vi "UHR-Fleezers Control (host) - 12.6.1.vi"() -> ()   [LabVIEW 2012] (continued)
  T22 = cluster{"New Image":T2, "New Image":T2, "New Image":T2, "New Image":T2, "New Image":T2}
  T23 = typedef "XDNodeRunTimeDep.lvlib/timing_clust.ctl" = cluster{"Expected End [f-1]":u64, "Actual End [f-1]":u64, "Finished Late? [f-1]":bool, "Expected End [i-1]":u64, "Actual End [i-1]":u64, "Finished Late? [i-1]":bool, "Expected Start [i]":u64, "Actual Start [i]":u64, "Expected Start [f]":u64, "Actual Start [f]":u64, "Source Name":string, "Structure Name":string, "Period":i64, "Deadline":i64, "Offset":i64, "Start":i64, "Priority":i32, "Timeout":i32, "Mode":T24, "Wakeup Reason":T25, "Error":errorcluster, "Source Type":string, "Secondary Source Type":string, "Global End Time":u64, "Global Start Time":u64, "Frame Duration":u64, "Iteration Duration":u64, "Assigned CPU":i32, "I/O Scan Engine Mode":u32}
  T24 = typedef "XDNodeRunTimeDep.lvlib/nitl_modes.ctl" = enum32{"No Change", "Process missed periods, maintain original phase", "Discard missed periods, maintain original phase", "Process missed periods, ignore original phase", "Discard missed periods, ignore original phase"}
  T25 = typedef "XDNodeRunTimeDep.lvlib/wakeup.ctl" = enum32{"Normal", "Aborted", "Asynchronous wakeup", "Timing source error", "Timed loop error", "Timeout"}
  T26 = enum32{"Status", "Sample Stage", "Syringe Pump", "Trap Control (RF)", "APD Counting", "Fluorescence Laser Control", "Trap AI", "Video", "FPGA"}
  T27 = enum32{"Status", "Sample Stage", "Syringe Pump", "Trap Control (RF)", "APD Counting", "Fluorescence Laser Control", "Trap AI", "Video", "FPGA", "Misc. Configuration"}
  T28 = enum16{"big-endian, network order", "native, host order", "little-endian"}
  T29 = enum16{"open", "replace", "create", "open or create", "replace or create", "replace or create with confirmation"}
  T30 = cluster{"Scan Range AOD (nm) 2":dbl, "Step Size AOD (nm) 2":dbl, "Scan Speed AOD (nm/s) 2":dbl, "Number of scans (AOD) 2":u16, "Label":string}
  T31 = cluster{"[0]":dbl, "[1]":dbl, "[2]":dbl, "[3]":dbl, "[4]":dbl, "[5]":dbl}
  T32 = cluster{"Diameter (mm)":dbl, "Units":dbl, "Volume":dbl, "Rate":dbl}
  T33 = cluster{"Left":i32, "Top":i32, "Width":u32, "Height":u32}
  T34 = cluster{cluster{"Left":i32, "Top":i32, "Width":u32, "Height":u32}}[]
  T35 = enum32{"Normal Display", "Dual Display (APD)", "FFT", "High Res Display"}
  T36 = cluster{"Origin Pixel":cluster{"X":sgl, "Y":sgl}, "Angle Relative to Horizontal (deg)":sgl, "Axis Reference":u32}
  T37 = typedef "Simple Grid Descriptor" = cluster{"X Step":sgl, "Y Step":sgl, "Unit":T38}
  T38 = typedef "Image Unit" = enum32{"Undefined", "Angström", "Micrometer", "Millimeter", "Centimeter", "Meter", "Kilometer", "Microinch", "Inch", "Feet", "Nautical miles", "Standard miles", "Steps"}
  T39 = cluster{"averaging mode":u16, "weighting mode":u16, "number of averages":u32}
  T40 = cluster{"dB On (F)":bool, "unwrap phase (F)":bool, "convert to degree (F)":bool}
  T41 = cluster{string, string, string, string, string, string, string, string}
  T42 = cluster{string, string, string, string, string, string, string, string, string, string, string, string}
  T43 = cluster{string, string, string, string, string, string, string, string, string, string, string, string, string}
  T44 = cluster{string, string, string, string, string, string, string, string, string, string, string, string, string, string}
  T45 = cluster{"BD 1 Frequency 1 (MHz)":dbl, "BD 1 Frequency 2 (MHz)":dbl}
  T46 = cluster{"f0":dbl, "df":dbl, "magnitude":dbl[]}[][]
  T47 = cluster{"Comment (data description)":string, "Channel 1 Buffer":string, "Channel 2 Buffer":string, "Channel 3 Buffer":string, "Title":string, "DNA Construct":string, "Bead diameter":dbl, "Name":string}
  T48 = enum32{"setting", "request", "request control", "info", "statistics", "system settings", "I/O sub system", "HRT control", "camera descriptions", "device specific data", "event sub system settings", "event sub system results", "image memory manager"}
  T49 = typedef "AviRefnum.ctl" = refnum<k1>
  T50 = typedef "imagedata.ctl" = cluster{"image type":i32, "image depth":i32, "image":u8[], "mask":u8[], "colors":u32[], "Rectangle":cluster{"left":i16, "top":i16, "right":i16, "bottom":i16}}
diagram:
  w7 = u16 10 items=["1.0"=10, "1.5"=15, "2.0"=20] ("stop bits (10: 1 bit)")
  w74 = u16 20 items=["1.0"=10, "1.5"=15, "2.0"=20] ("stop bits (10: 1 bit)")
  w77 = u16 20 items=["1.0"=10, "1.5"=15, "2.0"=20] ("stop bits (10: 1 bit)")
  w103 = u16 20 items=["1.0"=10, "1.5"=15, "2.0"=20] ("stop bits (10: 1 bit)")
  w13 = T18 2 items=["Grayscale (U8)", "Grayscale (I16)", "Grayscale (SGL)", "Complex (CSG)", "RGB (U32)", "HSL (U32)", "RGB (U64)", "Grayscale (U16)"] ("Image Type")
  w233 = 10.0 ("y")
  w232 = 32767.0 ("y")
  w248 = 6.0  # clock mult.
  w249 = 49152000.0  # TCXO frequ.
  # "What are these?"
  # "I don't think you need to do this.\nEverytime you want to adjust phase you always set this anyway.\nSince we removed the separate +/- controls.\n\nHaven't added for added fl lasers.  Should remove this code."
  # "Bottom 1 Harvard"
  # "Top 3 Harvard"
  # "Center Harvard"
  # "Bottom 1 Harvard"
  # "Top 3 Harvard"
  # "Center Harvard"
  n1 = Build Array("DIO count 1 (ticks)", "DIO count 2 (ticks)", "DIO count 3 (ticks)") -> (w154:u16[])
  n2 = xnode "Open FPGA VI Reference"("resource name"=T19 "750kHzDAQ") -> ("FPGA VI Reference Out"=w257:T20, "error out"=w256:errorcluster)  [unwired: 1 in]
  n3 = local read "AO1"() -> (w227:dbl)
  n4 = local read "AO2"() -> (w226:dbl)
  n5 = local read "Scan Increment (MHz)"() -> (w244:dbl)
  n6 = local read "Continuous MCL Scanning"() -> (w214:bool)
  n7 = local read "Fast Scan Dir"() -> (w213:bool)
  n8 = xnode "Invoke Method"("FPGA VI Reference In"=w257, "error in"=w256) -> ("FPGA VI Reference Out"=w17:T20, "error out"=w173:errorcluster)
  n9 = local read "Number of scans (MCL)"() -> (w215:u64)
  n10 = Multiply(x=w227, y=w232) -> (x*y=w229:dbl)
  n11 = Multiply(x=w226, y=w232) -> (x*y=w231:dbl)
  n12 = Divide(x=w229, y=w233) -> (x/y=w228:dbl)
  n13 = Divide(x=w231, y=w233) -> (x/y=w230:dbl)
  n14 = To Word Integer(number=w228) -> (16bit integer=w225:i16)
  n15 = To Word Integer(number=w230) -> (16bit integer=w224:i16)
  n16 = Not(x=w213) -> (.not. x?=w208:bool)
  n17 = local read "Cycles/step (MCL)"() -> (w216:u64)
  n18 = Multiply(x=w244, y=1000.0) -> (x*y=w251:dbl)
  n19 = local read "Scan steps (MCL)"() -> (w217:u64)
  n20 = local read "Desired Scan Incr (V)"() -> (w219:dbl)
  n21 = Scale By Power Of 2(n=48, x=w251) -> (x*2^n=w252:dbl)
  n22 = Unbundle By Name(cluster{"output high":i16, "output low":i16} {"output high"=3000, "output low"=0} ("FB output range 1")) -> ("output high"=w55:i16, "output low"=w54:i16)
  n23 = Multiply(x=w249, y=w248) -> (x*y=w247:dbl)
  n24 = Divide(x=w252, y=w247) -> (x/y=w246:dbl)
  n25 = local read "Setpoints (V)"() -> (w263:cluster{"Set 1":dbl, "Set 2":dbl})
  n26 = To Quad Integer(1:w246) -> (0:w243:i64)
  n27 = Divide(x=40000000.0, y="AI Count (ticks)") -> (x/y=w204:dbl)
  n28 = Multiply(x=w219, y=32767.0) -> (x*y=w221:dbl)
  n29 = local read "Trap Intensity PID Gains"() -> (w258:T9)
  n30 = local write "Trap Pos FIFO Timeout"(u16 0 ("Trap Pos FIFO Timeout")) -> ()
  n31 = local read "Number Interlace Sets"() -> (w147:u8)
  n32 = Split 1D Array(array=w154, index=w147) -> (first subarray=w156:u16[])  [unwired: 1 out]
  n33 = Add Array Elements(numeric array=w156) -> (sum=w155:u16)
  n34 = local read "# Samples/channel"() -> (w236:u32)
  n35 = local read "Number of F/B Scans (AOD)"() -> (w237:u16)
  n36 = local read "Not-Interlacing Set"() -> (w146:enum32{"Set 1", "Set 2", "Set 3"})
  n37 = To Unsigned Byte Integer(number=w146) -> (unsigned 8bit integer=w152:u8)
  n38 = Index Array(array=w154, index=w152) -> (element=w153:u16)
  n39 = local read "Feedback On/Off"() -> (w266:cluster{"Set 1":bool, "Set 2":bool})
  n40 = local read "Scan steps (AOD)"() -> (w242:u64)
  n41 = local read "All FB On/Off"() -> (w267:bool)
  n42 = local read "Cycles/step (AOD)"() -> (w241:u64)
  n43 = local write "AI rate (Hz)"(w204) -> ()
  n44 = Divide(x=w221, y=10.0) -> (x/y=w220:dbl)
  n45 = Multiply(x=w242, y=w241) -> (x*y=w240:u64)
  n46 = Unbundle By Name(w258) -> ("proportional gain (Kc)"=w59:i16, "integral gain (Kc*Ts/Ti)"=w58:i16, "derivative gain (Kc*Td/Ts)"=w57:i16)
  n47 = property on="AI Count (ticks)" class="DigNum (strict)"("Val(Sgnl)"="AI Count (ticks)") -> ()  [unwired: 2 in, 2 out]
  n48 = Multiply(x=3276.7, y=w263) -> (x*y=w262:cluster{"Set 1":dbl, "Set 2":dbl})
  n49 = To Word Integer(number=w220) -> (16bit integer=w218:i16)
  n50 = Multiply(x=w240, y=u64 2) -> (x*y=w238:u64)
  n51 = Divide(x=w204, y="FPGA Ave.") -> (x/y=w205:dbl)
  n52 = To Word Integer(number=w262) -> (16bit integer=w261:cluster{"Set 1":i16, "Set 2":i16})
  n53 = Multiply(x=w238, y=w237) -> (x*y=w235:u64)
  n54 = local read "Sets to FIFO (Traps)"() -> (w63:T15)
  n55 = local write "Ave. Rate (Hz)"(w205) -> ()
  n56 = Divide(x=w235, y=w236) -> (x/y=w234:dbl)
  n57 = Unbundle By Name(w261) -> ("Set 1"=w260:i16, "Set 2"=w259:i16)
  n58 = local read "2D or 1D Scan"() -> (w165:bool)
  n59 = local write "Data points/scans"(w235) -> ()
  n60 = local read "Scan BD"() -> (w253:bool)
  n61 = And(x=w266, y=w267) -> (x .and. y?=w265:cluster{"Set 1":bool, "Set 2":bool})
  n62 = local write "Data points/scan (f/b)"(w238) -> ()
  n63 = Reciprocal(x=w205) -> (1/x=w206:dbl)
  n64 = local read "N Acq Sets (Traps + Fl.)"() -> (w197:i16)
  n65 = local write "N sets should be saved"(w234) -> ()
  n66 = Unbundle By Name(w265) -> ("Set 1"=w269:bool, "Set 2"=w268:bool)
  n67 = local read "Interlace"() -> (w148:bool)
  n68 = Select(t=w155, s=w148, f=w153) -> (s? t:f=w145:u16)
  n69 = local write "Update Count (MCL)"(w145) -> ()
  n70 = local write "Total Counts (ticks)"(w145) -> ()
  n71 = local write "Ave. Period (s)"(w206) -> ()
  n72 = Unbundle By Name(w63) -> ("Set 1"=w62:bool, "Set 2"=w61:bool, "Set 3"=w60:bool)
  n73 = property on="2D or 1D Scan" class="Bool (strict)"("Val(Sgnl)"=w165) -> ()  [unwired: 2 in, 2 out]
  n74 = xnode "Read/Write Control"("FPGA VI Reference In"=w164, "error in"=w173, "ai count"="AI Count (ticks)", "Interlace ON/OFF"=w148, "Number Interlace Cycles"=w147, "Set 1"=w62, "Set 2"=w61, "Set 3"=w60, "FB On/Off Set 1"=w269, "FB On/Off Set 2"=w268, "Interlace Off Parameters"=w146, "FB Setpoint Set 1"=w260, "FB Setpoint Set 2"=w259, "P1"=w59, "I1"=w58, "D1"=w57, "FB1 output high"=w55, "FB1 output low"=w54, "Cycles per step"=w241, "Scan BD"=w253, "Number of scans"=w237, "Scan steps"=w242, "Scan freq.  increment"=w243, "AO1"=w225, "AO2"=w224, "Scan freq.  increment (MCL)"=w218, "Scan steps (MCL)"=w217, "Cycles per step (MCL)"=w216, "Number of scans (MCL)"=w215, "MCL count"=w145, "Cont. Scan (MCL)"=w214, "MCL Scan Axis"=w208, "1D or 2D Scan?"=w165, "N of AI1 Int Acq Sets"=w197, "Amp switch delay"="Amp switch delay", "Swap F1 and F2"="Swap F1 and F2", "APD to FIFO"=FALSE, "DIO count 1 (ticks)"="DIO count 1 (ticks)", "DIO count 2 (ticks)"="DIO count 2 (ticks)", "DIO count 3 (ticks)"="DIO count 3 (ticks)") -> ("FPGA VI Reference Out"=w19:T20, "error out"=w18:errorcluster)  [unwired: 1 in]
  n75 = local read "Laser interlacing mode"() -> (w144:enum32{"Laser ON", "Laser OFF", "Interlace"})
  n76 = local read "Green Laser ON"() -> (w143:bool)
  n77 = local read "Trap Pos. FB Range"() -> (w53:T12)
  n78 = local read "Trap Pos. FB Gains"() -> (w52:T11)
  n79 = Multiply(x="Green Intensity % (FB OFF)", y=655.35) -> (x*y=w136:dbl)
  n80 = local read "Invert laser interlacing"() -> (w32:bool)
  n81 = local read "Trap Pos. AI1 X Pre-scale"() -> (w91:u16)
  n82 = Multiply(x="Green FB Setpoint (mV)", y=3.2767) -> (x*y=w133:dbl)
  n83 = local read "Trap Pos FB Int Count"() -> (w85:u16)
  n84 = local read "Differential FB?"() -> (w79:bool)
  n85 = local read "Neg. TTrig FPGA"() -> (w81:bool)
  n86 = Multiply(x="Red FB Setpoint (mV)", y=3.2767) -> (x*y=w40:dbl)
  n87 = To Unsigned Word Integer(number=w136) -> (unsigned 16bit integer=w134:u16)
  n88 = Multiply(x="Red Intensity % (FB OFF)", y=655.35) -> (x*y=w36:dbl)
  n89 = To Word Integer(number=w133) -> (16bit integer=w131:i16)
  n90 = Unbundle By Name("Green FB Gains") -> ("proportional gain (Kc)"=w44:i16, "integral gain (Kc*Ts/Ti)"=w43:i16, "derivative gain (Kc*Td/Ts)"=w42:i16)
  n91 = Unbundle By Name("Red FB Gains") -> ("proportional gain (Kc)"=w29:i16, "integral gain (Kc*Ts/Ti)"=w28:i16, "derivative gain (Kc*Td/Ts)"=w27:i16)
  n92 = case shown="False" w143 {
    tunnel: w144 -> [_ w295]
    tunnel: [enum32{"Laser ON", "Laser OFF", "Interlace"}."Laser OFF" ("Green laser mode") w295] -> w31
    frame False {
    }
    frame True {
    }
  }
  n93 = To Word Integer(number=w40) -> (16bit integer=w37:i16)
  n94 = Unbundle By Name(w52) -> ("proportional gain (Kc)"=w48:fxp<+/-,16,8>, "integral gain (Kc*Ts/Ti)"=w47:fxp<+/-,16,8>, "derivative gain (Kc*Td/Ts)"=w46:fxp<+/-,16,8>)
  n95 = To Unsigned Word Integer(number=w36) -> (unsigned 16bit integer=w33:u16)
  n96 = Unbundle By Name(w53) -> ("output high"=w51:fxp<+/-,16,1>, "output low"=w49:fxp<+/-,16,1>)
  n97 = local read "Trap Pos FB Monitor\nT1 or T2"() -> (w96:bool)
  n98 = local read "Trap Pos FB Negate Action"() -> (w95:bool)
  n99 = local read "Trap Pos. FB Offset Factor"() -> (w94:i64)
  n100 = local read "Trap Pos. FB Mult Factor"() -> (w93:i64)
  n101 = xnode "Read/Write Control"("FPGA VI Reference In"=w19, "error in"=w18, "Invert GI 2"=w32, "Operating Mode 2"=w31, "P3"=w44, "I3"=w43, "D3"=w42, "Green FB Setpoint"=w131, "Green FB On/Off"="Green FB On/Off", "Current Out"=w134, "Green int current ON count adj"="Green int current ON count adj", "Operating Mode"=w31, "Invert GI"=w32, "Trap Pos FB Monitor T1 or T2"=w96, "Trap Pos FB Negate Action"=w95, "Trap Pos. FB Offset Factor"=w94, "Trap Pos. FB Mult Factor"=w93, "Force feedback"=FALSE, "AI1 X Scale"=w91, "Trap Pos to FIFO"=TRUE, "Trap Pos FB Int Count"=w85, "TTrig Negate Pos"=w81, "FB Trig Integrate"="FB Trig Integrate", "Diff FB Measurement?"=w79, "Negate Diff?"="Negate Diff?", "P2"=w48, "I2"=w47, "D2"=w46, "FB2 output high"=w51, "FB2 output low"=w49, "Red FB Setpoint"=w37, "RI Current Out"=w33, "Red Laser Operating Mode"=w31, "RI Operating Mode 2"=w31, "Invert RI 2"=w32, "Invert RI"=w32, "P4"=w29, "I4"=w28, "D4"=w27, "Red FB On/Off"="Red FB On/Off") -> ("FPGA VI Reference Out"=w23:T20, "error out"=w25:errorcluster)
  n102 = stacked-sequence {
    tunnel: w25 -> [_ _ _ w306]
    tunnel: [_ _ _ w306] -> w24
    tunnel: w23 -> [_ _ _ w307]
    tunnel: [_ _ _ w307] -> w22
    frame #0 {
      w296 = T21."empty" ("mode")
      # "Clear external fluorescence triggering FIFO"
      # "APD loop counts"
      # "Fluorescence loop counts (rates)"
      n103 = local read "APD Integration Time (s)"() -> (w298:dbl)
      n104 = local read "Interlace ON count"() -> (w299:u16)
      n105 = call "Smart Buffer (DBL) 1.vi"("mode"=w296) -> ()  [unwired: 5 in, 6 out]
      n106 = call "Smart Buffer (DBL) 2.vi"("mode"=w296) -> ()  [unwired: 5 in, 6 out]
      n107 = property on="APD Integration Time (s)" class="DigNum (strict)"("Val(Sgnl)"=w298) -> ()  [unwired: 2 in, 2 out]
      n108 = property on="Interlace ON count" class="DigNum (strict)"("Val(Sgnl)"=w299) -> ()  [unwired: 2 in, 2 out]
      "Number of APDs" <- 3.0 ("Number of APDs")
    }
    frame #1 {
      # "Number of APDs affects\nAPD DMA transfer"
      # "General settings for all lasers:"
      # "And includes all laser\nON/OFF settings"
      # "Fluorescent lasers settings:"
      # "Blue laser settings:"
      n109 = local read "Laser interlacing mode"() -> (w301:enum32{"Laser ON", "Laser OFF", "Interlace"})
      n110 = local read "Invert laser interlacing"() -> (w300:bool)
      n111 = local read "Blue FB On/Off"() -> (w302:bool)
      n112 = property on="Blue FB On/Off" class="Bool (strict)"("Val(Sgnl)"=w302) -> ()  [unwired: 2 in, 2 out]
      n113 = property on="Invert laser interlacing" class="Bool (strict)"("Val(Sgnl)"=w300) -> ()  [unwired: 2 in, 2 out]
      n114 = property on="Laser interlacing mode" class="RadioBtnsControl (strict)"("Val(Sgnl)"=w301) -> ()  [unwired: 2 in, 2 out]
    }
    frame #2 {
      w303 = path "C:/Home/wheeler/Comstock-LabView-Link.udl" ("connection information")
      # "Initialize the database connection"
      n115 = call-poly <vilib>:"DB Tools Open Connection.vi"("connection information"=w303) -> ("connection reference"=w304:T17)  [unwired: 7 in, 1 out]
      "connection reference" <- w304
      n116 = local write "connection reference"(w304) -> ()
      n117 = local write "Database link"(w303) -> ()
    }
    frame #3 {
      n118 = Wait (ms)(milliseconds to wait=u32 1000) -> ()  [unwired: 1 out]
    }
  }
  n119 = local write "Offset (nm)"(0.0 ("Offset (nm)")) -> ()
  n120 = local write "Bead Mean (nm)"(0.0 ("Bead Mean (nm)")) -> ()
  n121 = case shown="\"1axis\", Default" "1axis AOM vs 2 axis AOD" {
    tunnel: [T16 {"Minimum"=0.0, "Maximum"=40.0, "Increment"=1.0} ("Min Max Inc") T16 {"Minimum"=60.0, "Maximum"=90.0, "Increment"=1.0} ("Min Max Inc")] -> w4
    tunnel: [T16 {"Minimum"=0.0, "Maximum"=45.0, "Increment"=1.0} ("Data Entry Limits") T16 {"Minimum"=0.0, "Maximum"=50.0, "Increment"=1.0} ("Data Entry Limits")] -> w2
    frame "2axisAOD" {
      # "Amp Limits"
      # "Freq Limits"
      n122 = local write "Initial Phase Adjustment (DIO)"(160 ("Initial Phase Adjustment (DIO)")) -> ()
    }
    frame "1axis", Default {
      # "Amp Lmits"
      # "Freq Limits"
      n123 = local write "Initial Phase Adjustment (DIO)"(0 ("Initial Phase Adjustment (DIO)")) -> ()
    }
  }
  n124 = xnode "Invoke Method"("FPGA VI Reference In"=w22, "error in"=w24, "Requested Depth"="Trap AI FIFO Depth") -> ("FPGA VI Reference Out"=w99:T20, "error out"=w98:errorcluster)  [unwired: 1 out]
  n125 = xnode "Invoke Method"("FPGA VI Reference In"=w99, "error in"=w98, "Requested Depth"="Trap Position FIFO Depth") -> ("FPGA VI Reference Out"=w87:T20, "error out"=w86:errorcluster)  [unwired: 1 out]
  n126 = flat-sequence "Safety limits on RF frequencies and amplitudes (for AOM protection)" {
    tunnel: w17 -> [w318]
    tunnel: [w318] -> w164
    tunnel: [w315] -> w163
    tunnel: [w314] -> w162
    tunnel: [w316] -> w160
    tunnel: [w317] -> w161
    tunnel: w4 -> [w315]
    tunnel: w2 -> [w314]
    frame #0 {
      w317 = T16 {"Minimum"=0.0, "Maximum"=40.0, "Increment"=1.0} ("Min Max Inc")
      w316 = T16 {"Minimum"=0.0, "Maximum"=45.0, "Increment"=1.0} ("Data Entry Limits")
      n127 = property on="BD 2 Frequency 1 (MHz)" class="DigNum (strict)"("Data Range"=w317) -> ()  [unwired: 2 in, 2 out]
      n128 = property on="BD 2 Frequency 3 (MHz)" class="DigNum (strict)"("Data Range"=w317) -> ()  [unwired: 2 in, 2 out]
      n129 = property on="BD 2 Frequency 2 (MHz)" class="DigNum (strict)"("Data Range"=w317) -> ()  [unwired: 2 in, 2 out]
      n130 = property on="BD 1 Frequency 1 (MHz)" class="DigNum (strict)"("Data Range"=w315) -> ()  [unwired: 2 in, 2 out]
      n131 = property on="BD 1 Frequency 2 (MHz)" class="DigNum (strict)"("Data Range"=w315) -> ()  [unwired: 2 in, 2 out]
      n132 = property on="BD 1 Frequency 3 (MHz)" class="DigNum (strict)"("Data Range"=w315) -> ()  [unwired: 2 in, 2 out]
      n133 = property on="BD 2 Amplitude 1 (%)" class="DigNum (strict)"("Data Range"=w316) -> ()  [unwired: 2 in, 2 out]
      n134 = property on="BD 2 Amplitude 2 (%)" class="DigNum (strict)"("Data Range"=w316) -> ()  [unwired: 2 in, 2 out]
      n135 = property on="BD 2 Amplitude 3 (%)" class="DigNum (strict)"("Data Range"=w316) -> ()  [unwired: 2 in, 2 out]
      n136 = property on="BD 1 Amplitude 3 (%)" class="DigNum (strict)"("Data Range"=w314) -> ()  [unwired: 2 in, 2 out]
      n137 = property on="BD 1 Amplitude 2 (%)" class="DigNum (strict)"("Data Range"=w314) -> ()  [unwired: 2 in, 2 out]
      n138 = property on="BD 1 Amplitude 1 (%)" class="DigNum (strict)"("Data Range"=w314) -> ()  [unwired: 2 in, 2 out]
      "X RF Frequency Limits (MHz)" <- w315
      "X RF Amplitude Limits (%)" <- w314
      "Y RF Amplitude Limits (%)" <- w316
      "Y RF Frequency Limits (MHz)" <- w317
    }
  }
  n139 = xnode "Invoke Method"("FPGA VI Reference In"=w87, "error in"=w86) -> ("FPGA VI Reference Out"=w172:T20, "error out"=w171:errorcluster)  [unwired: 1 in]
  n140 = flat-sequence "Initial FPGA Loop Relative Phase Adjustment" {
    tunnel: "Initial Phase Adjustment (AI1)" -> [w334]
    tunnel: "Initial Phase Adjustment (GI)" -> [w333]
    tunnel: w172 -> [w332]
    tunnel: w171 -> [w331]
    tunnel: "Initial Phase Adj. (MCL)" -> [w330]
    tunnel: [w335] -> w181
    tunnel: [w329] -> w177
    tunnel: "Initial Phase Adjustment (APD Acq)" -> [w328]
    tunnel: "Initial Phase Adjustment (APD 1 Gate)" -> [w327]
    tunnel: "Initial Phase Adjustment (Green FB)" -> [w326]
    tunnel: "Initial Phase Adjustment (GI) 2" -> [w325]
    tunnel: "Initial Phase Adjustment (APD 2 Gate)" -> [w324]
    tunnel: "Initial Phase Adjustment (RI)" -> [w323]
    tunnel: "Initial Phase Adjustment (BI DO)" -> [w322]
    tunnel: "Initial Phase Adjustment (BI AO)" -> [w321]
    tunnel: "Initial Phase Adjustment (APD 3 Gate)" -> [w320]
    tunnel: "Initial Phase Adjustment (DIO)" -> [w319]
    tunnel: w181 -> [w337]
    tunnel: [w338] -> w178
    tunnel: w177 -> [w338]
    tunnel: [w337] -> w176
    tunnel: w178 -> [w341]
    tunnel: w176 -> [w340]
    tunnel: [w343] -> w175
    tunnel: [w342] -> w174
    tunnel: [w345] -> w179
    tunnel: [w346] -> w180
    tunnel: w175 -> [w346]
    tunnel: w174 -> [w345]
    frame #0 {
      n141 = xnode "Read/Write Control"("FPGA VI Reference In"=w332, "error in"=w331, "Phase count adjustment"=w334, "Phase count adjustment (GI)"=w333, "Phase count adjustment (MCL)"=w330, "Phase Count Adjustment (APD Acq)"=w328, "Phase count adjustment (APD 1 Gate)"=w327, "Phase count adjustment (APD 2 Gate)"=w324, "Phase count adjustment (Green FB)"=w326, "Phase count adjustment (GI) 2"=w325, "Phase count adjustment (RI)"=w323, "Phase count adjustment (BI AO)"=w321, "Phase count adjustment (BI D)"=w322, "Phase count adjustment (APD 3 Gate)"=w320, "Phase count adjustment (DIO)"=w319) -> ("FPGA VI Reference Out"=w329:T20, "error out"=w335:errorcluster)
    }
    frame #1 {
      n142 = Wait (ms)(milliseconds to wait=u32 100) -> ()  [unwired: 1 out]
    }
    frame #2 {
      w339 = TRUE
      n143 = xnode "Read/Write Control"("FPGA VI Reference In"=w341, "error in"=w340, "+ phase"=w339, "+ phase (GI)"=w339, "+ phase (MCL)"=w339, "+ phase (APD Acq)"=w339, "+ phase (APD 1 Gate)"=w339, "+ phase (APD 2 Gate)"=w339, "+ phase (Green FB)"=w339, "+ phase (GI) 2"=w339, "+ phase (RI)"=w339, "+ phase (BI AO)"=w339, "+ phase (BI D)"=w339, "+ phase (APD 3 Gate)"=w339, "+ phase (DIO)"=w339) -> ("FPGA VI Reference Out"=w342:T20, "error out"=w343:errorcluster)
    }
    frame #3 {
      n144 = Wait (ms)(milliseconds to wait=u32 100) -> ()  [unwired: 1 out]
    }
  }
  n145 = local read "Phase adj. (Green FB)"() -> (w157:i16)
  n146 = local read "Phase adj. (GI) 2"() -> (w137:i16)
  n147 = local read "Phase adjust (MCL)"() -> (w209:i16)
  n148 = local read "Phase adj. (AI1)"() -> (w211:i16)
  n149 = local read "Phase adj. (GI)"() -> (w210:i16)
  n150 = xnode "Read/Write Control"("FPGA VI Reference In"=w179, "error in"=w180, "Phase count adjustment"=w211, "Phase count adjustment (GI)"=w210, "Phase count adjustment (MCL)"=w209, "Phase Count Adjustment (APD Acq)"="Phase Adj. (APD Acq)", "Phase count adjustment (APD 1 Gate)"="Phase Adj. (APD 1 Gate)", "Phase count adjustment (APD 2 Gate)"="Phase Adj. (APD 2 Gate)", "Phase count adjustment (Green FB)"=w157, "Phase count adjustment (GI) 2"=w137) -> ("FPGA VI Reference Out"=w123:T20, "error out"=w186:errorcluster)
  n151 = call "Initialize RF boards - interlace 3.vi"("error in"=w186, "FPGA VI Reference In"=w123) -> ("error out"=w184:errorcluster, "FPGA VI Reference Out"=w185:T20)
  n152 = call "set RF board frequency - interlace.vi"("Board 2 Frequency Limits"=w161, "Board 1 Frequency Limits"=w163, "error in"=w184, "FPGA VI Reference In"=w185, "Board 2 Frequency 3 (MHz)"="BD 2 Frequency 3 (MHz)", "Board 1 Frequency 3 (MHz)"="BD 1 Frequency 3 (MHz)", "Board 2 Frequency 2 (MHz)"="BD 2 Frequency 2 (MHz)", "Board 2 Frequency 1 (MHz)"="BD 2 Frequency 1 (MHz)", "Board 1 Frequency 2 (MHz)"="BD 1 Frequency 2 (MHz)", "Board 1 Frequency 1  (MHz)"="BD 1 Frequency 1 (MHz)") -> ("error out"=w284:errorcluster, "FPGA VI Reference Out"=w285:T20)
  n153 = call "set RF board amplitude - interlace.vi"("Board 2 Amplitude Limits"=w160, "Board 1 Amplitude Limits"=w162, "error in"=w284, "FPGA VI Reference In"=w285, "Board 2 Amplitude 3 (%)"="BD 2 Amplitude 3 (%)", "Board 1 Amplitude 3 (%)"="BD 1 Amplitude 3 (%)", "Board 2 Amplitude 2 (%)"="BD 2 Amplitude 2 (%)", "Board 2 Amplitude 1 (%)"="BD 2 Amplitude 1 (%)", "Board 1 Amplitude 2 (%)"="BD 1 Amplitude 2 (%)", "Board 1 Amplitude 1 (%)"="BD 1 Amplitude 1 (%)") -> ("error out"=w272:errorcluster, "FPGA VI Reference Out"=w273:T20)
  n154 = flat-sequence {
    tunnel: w273 -> [w356]
    tunnel: w272 -> [w355]
    tunnel: [w354] -> w277
    tunnel: [w353] -> w276
    tunnel: [w360] -> w275
    tunnel: w277 -> [w360]
    tunnel: [w359] -> w274
    tunnel: w276 -> [w359]
    tunnel: w275 -> [w369]
    tunnel: w274 -> [w368]
    tunnel: [w367] -> w16
    tunnel: [w366] -> w88
    frame #0 {
      w347 = FALSE ("Retract Pump 3")
      n155 = local read "Trap 1 (ON/OFF)"() -> (w348:bool)
      n156 = xnode "Read/Write Control"("FPGA VI Reference In"=w356, "error in"=w355, "Direct RF Box  Communication"=FALSE) -> ("FPGA VI Reference Out"=w354:T20, "error out"=w353:errorcluster)
      n157 = local write "Saving..."(FALSE ("Saving Data")) -> ()
      n158 = local write "Stop All"(FALSE ("Stop All")) -> ()
      n159 = local write "Retract Pump 1"(w347) -> ()
      n160 = local write "Retract Pump 3"(w347) -> ()
      n161 = local write "Index"(1.0 ("Index")) -> ()
      n162 = property on="Trap 1 ON" class="Bool (strict)"("Value"=w348) -> ()  [unwired: 2 in, 2 out]
      "Manipulating Trap" <- FALSE ("Manipulating Trap")
    }
    frame #1 {
      n163 = local read "Trap 2 (ON/OFF)"() -> (w358:bool)
      n164 = Wait (ms)(milliseconds to wait=u32 10) -> ()  [unwired: 1 out]
      n165 = property on="Trap 2 ON" class="Bool (strict)"("Val(Sgnl)"=w358) -> ()  [unwired: 2 in, 2 out]
    }
    frame #2 {
      n166 = local read "Scan Range (nm)"() -> (w362:dbl)
      n167 = xnode "Read/Write Control"("FPGA VI Reference In"=w369, "error in"=w368, "FPGA Controls  RF Box"=TRUE ("Direct RF Box  Communication")) -> ("FPGA VI Reference Out"=w367:T20, "error out"=w366:errorcluster)
      n168 = call "Update messages.vi"("Message to add"="UHR-Fleezers ready.", "Old message string"="") -> ("New message string"=w365:string)
      n169 = local write "Messages"(w365) -> ()
      n170 = property on="Scan Range (nm)" class="DigNum (strict)"("Val(Sgnl)"=w362) -> ()  [unwired: 2 in, 2 out]
    }
  }
  n171 = Subtract(x="BD 1 Frequency 1 (MHz)", y="BD 1 Frequency 2 (MHz)") -> (x-y=w196:dbl)
  n172 = Subtract(x="BD 2 Frequency 1 (MHz)", y="BD 2 Frequency 2 (MHz)") -> (x-y=w195:dbl)
  n173 = Square(x=w195) -> (x^2=w193:dbl)
  n174 = Square(x=w196) -> (x^2=w194:dbl)
  n175 = Add(x=w194, y=w193) -> (x+y=w192:dbl)
  n176 = Square Root(x=w192) -> (sqrt(x)=w191:dbl)
  n177 = local write "Trap Delta (MHz)"(w191) -> ()
  n178 = call-poly "VISA Configure Serial Port"("VISA resource name"="VISA resource name", "baud rate (9600)"=u32 115200, "stop bits (10: 1 bit)"=w7) -> ("VISA resource name out"=w6:refnum<visa-resource-name>, "error out"=w5:errorcluster)  [unwired: 4 in, 7 out]
  n179 = call-poly "VISA Configure Serial Port"("VISA resource name"="Bottom  1 Harvard Syringe Pump Serial Port", "baud rate (9600)"=u32 115200, "stop bits (10: 1 bit)"=w74) -> ("VISA resource name out"=w70:refnum<visa-resource-name>, "error out"=w69:errorcluster)  [unwired: 4 in, 7 out]
  n180 = call-poly "VISA Configure Serial Port"("VISA resource name"="Top 3 Harvard Syringe Pump Serial Port", "baud rate (9600)"=u32 115200, "stop bits (10: 1 bit)"=w77) -> ("VISA resource name out"=w72:refnum<visa-resource-name>, "error out"=w71:errorcluster)  [unwired: 4 in, 7 out]
  n181 = call-poly "VISA Configure Serial Port"("VISA resource name"="Sample Chamber Stage Serial Port") -> ("VISA resource name out"=w118:refnum<visa-resource-name>, "error out"=w119:errorcluster)  [unwired: 5 in, 8 out]
  "Stage Control Serial Error" <- w119
  n182 = local write "Blue Error Out"(w5) -> ()
  n183 = call-poly "VISA Configure Serial Port"("VISA resource name"="Center Harvard Syringe Pump Serial Port", "baud rate (9600)"=u32 115200, "stop bits (10: 1 bit)"=w103) -> ("VISA resource name out"=w100:refnum<visa-resource-name>, "error out"=w101:errorcluster)  [unwired: 4 in, 7 out]
  n184 = call "IMAQ Create"("Image Name"="APD 1 Image", "Image Type"=w13) -> ("New Image"=w109:T2)  [unwired: 3 in, 1 out]
  n185 = call "IMAQ Create"("Image Name"="APD 2 Image", "Image Type"=w13) -> ("New Image"=w108:T2)  [unwired: 3 in, 1 out]
  n186 = call "IMAQ Create"("Image Name"="APD 3 Image", "Image Type"=w13) -> ("New Image"=w12:T2)  [unwired: 3 in, 1 out]
  n187 = call "IMAQ Create"("Image Name"="Det. X Image", "Image Type"=w13) -> ("New Image"=w107:T2)  [unwired: 3 in, 1 out]
  n188 = call "IMAQ Create"("Image Name"="Det. Y Image", "Image Type"=w13) -> ("New Image"=w106:T2)  [unwired: 3 in, 1 out]
  n189 = Bundle("New Image"=w109, "New Image"=w108, "New Image"=w12, "New Image"=w107, "New Image"=w106) -> (w105:T22)  [unwired: 1 in]
  n190 = node-c288() -> (w114:T23)  [unwired: 4 in]
  n191 = node-c288(3 ("Processor")) -> (w125:T23)  [unwired: 3 out]
  n192 = node-c288(2 ("Processor")) -> (w127:T23)  [unwired: 3 out]
  n193 = node-c288() -> (w129:T23)  [unwired: 4 out]
  n194 = node-c288(i64 1 ("Period"), 1 ("Processor")) -> (w200:T23)  [unwired: 2 out]
  n195 = timed-loop "Run Scripts, including: stage motion" {
    tunnel: w119 -> [w378]
    tunnel: w118 -> [w379]
    tunnel: [w379] -> w117
    tunnel: [w378] -> w116
    timing: w114 -> [_]
    timing-out: [_] -> w113
    tunnel: w100 -> [w377]
    tunnel: w101 -> [w376]
    tunnel: w72 -> [w373]
    tunnel: w71 -> [w372]
    tunnel: w70 -> [w374]
    tunnel: w69 -> [w375]
    tunnel: w6 -> [w371]
    stop <- w380 stop-if-true
    n196 = node-c288() -> ()  [unwired: 1 in, 1 out]
    n197 = event shown="[6] \"Move in a Circle\": Value Change" {
      selector: _ -> [_ _ _ _ _ _ _ _ _ _ _ _ _ _ _ _ _ _ _ _ _ _ _ _]
      dyn-events: _ -> [_ _ _ _ _ _ _ _ _ _ _ _ _ _ _ _ _ _ _ _ _ _ _ _]
      timeout: _ -> [_ _ _ _ _ _ _ _ _ _ _ _ _ _ _ _ _ _ _ _ _ _ _ _]
      tunnel: ["Set Position" "Move to Position" _ _ _ _ _ _ _ "Read Harvard" _ _ _ _ _ _ "Got ADig bead" "Force FB Data\nScript" _ "Got DNA bead" "Take Stepping Data" _ "Take Detection Laser\nImage" _] -> _
      tunnel: [_ _ _ _ _ _ _ _ _ _ _ _ _ _ _ _ _ _ _ _ _ _ _ w1118] -> w380
      tunnel: w378 -> [w398 w406 w419 w449 _ _ _ _ _ _ w609 w649 w730 w759 w891 w917 _ w953 _ _ _ _ _ _]
      tunnel: w379 -> [w399 w407 w420 w450 _ _ _ _ _ _ w610 w650 w731 w760 w892 w918 _ w954 _ _ _ _ _ _]
      tunnel: w377 -> [_ _ _ _ _ _ _ _ _ w594 _ _ _ _ _ _ _ _ _ _ _ _ _ _]
      tunnel: w376 -> [_ _ _ _ _ _ _ _ _ w593 _ _ _ _ _ _ _ _ _ _ _ _ _ _]
      tunnel: w375 -> [_ _ _ _ _ _ _ _ _ _ _ _ _ _ _ _ _ _ _ _ _ _ _ _]
      tunnel: w374 -> [_ _ _ _ _ _ _ _ _ _ _ _ _ _ _ _ _ _ _ _ _ _ _ _]
      tunnel: w373 -> [_ _ _ _ _ _ _ _ _ _ _ _ _ _ _ _ _ _ _ _ _ _ _ _]
      tunnel: w372 -> [_ _ _ _ _ _ _ _ _ _ _ _ _ _ _ _ _ _ _ _ _ _ _ _]
      tunnel: w371 -> [_ _ _ _ w477 w505 _ w573 w584 _ _ _ _ _ _ _ _ _ _ _ _ _ _ w1117]
      event "Set Position", "Set Position 2", "Set Position 3", "Set Position 4", "Set Position 5", "Set Position 1": Value Change {
        n198 = event-data() -> ()  [unwired: 1 in, 5 out]
        n199 = Build Array("Set Position 1", "Set Position 2", "Set Position 3", "Set Position 4", "Set Position 5") -> (w397:bool[])
        n200 = Boolean Array To Number(Boolean array=w397) -> (number=w396:u32)
        n201 = Logarithm Base 2(1:w396) -> (0:w388:dbl)
        n202 = call "Read Stage Position.vi"("error in"=w398, "VISA resource name in"=w399) -> ("Current Position"=w403:cluster{dbl, dbl, dbl}, "error out"=w402:errorcluster)  [unwired: 2 out]
        n203 = Decrement(x="Position") -> (x-1=w386:dbl)
        n204 = Greater Or Equal?(x=w388, y=0.0) -> (x >= y?=w389:bool)
        n205 = Cluster To Array(cluster=w403) -> (array=w400:dbl[])
        n206 = local write "Stage Control Serial Error"(w402) -> ()
        n207 = Select(t=w388, s=w389, f=w386) -> (s? t:f=w385:dbl)
        n208 = Increment(x=w385) -> (x+1=w384:dbl)
        n209 = Build Array (concatenate)(w384, w400) -> (w383:dbl[])
        n210 = Replace Array Subset(array="Saved Stage Positions", new element=w383, index (row)=w385) -> (w401:dbl[][])  [unwired: 1 in]
        n211 = local write "Saved Stage Positions"(w401) -> ()
      }
      event "Move to Position": Value Change {
        n212 = event-data() -> ()  [unwired: 1 in, 5 out]
        n213 = flat-sequence {
          tunnel: w407 -> [w411]
          tunnel: w406 -> [w410]
          frame #0 {
            n214 = local read "Saved Stage Positions"() -> (w413:dbl[][])
            n215 = local read "Position"() -> (w412:dbl)
            n216 = local write "Stage Moving"(TRUE ("Stage Moving")) -> ()
            n217 = call "move to saved stage position.vi"("error in"=w410, "Stage VISA resource name in"=w411, "Position"=w412, "Saved Stage Positions"=w413) -> ("error out"=w409:errorcluster)  [unwired: 1 out]
            n218 = local write "Stage Control Serial Error"(w409) -> ()
          }
          frame #1 {
            n219 = call <vilib>:"Beep.vi"() -> ()  [unwired: 3 in, 9 out]
            n220 = local write "Stage Moving"(FALSE ("Stage Moving")) -> ()
          }
        }
      }
      event "Move Cap. 1 (DNA Bottom)": Value Change {
        n221 = event-data() -> ()  [unwired: 1 in, 5 out]
        n222 = local write "Move Cap. 1 (DNA Bottom)"(FALSE ("Move Cap. 1 (DNA Right)")) -> ()
        n223 = flat-sequence {
          tunnel: w419 -> [w422]
          tunnel: w420 -> [w423]
          tunnel: [w423] -> w417
          tunnel: [w422] -> w416
          tunnel: w417 -> [w425]
          tunnel: w416 -> [w424]
          frame #0 {
            n224 = property on="Sample Channel\nFlow" class="Bool (strict)"("Val(Sgnl)"="Cap 1 Samp Flow ON") -> ()  [unwired: 2 in, 2 out]
          }
          frame #1 {
            n225 = local read "Saved Stage Positions"() -> (w435:dbl[][])
            n226 = local write "Stage Moving"(TRUE ("Stage Moving")) -> ()
            n227 = Array Subset(array=w435, index (row)=0 ("index"), length (row)=1 ("length"), index (col)=1 ("index"), length (col)=3 ("length")) -> (w432:dbl[][])
            n228 = Reshape Array(w432, 3 ("dimension size")) -> (w430:dbl[])
            n229 = Array To Cluster(array=w430) -> (cluster=w429:cluster{"[0]":dbl, "[1]":dbl, "[2]":dbl})
            n230 = call "Set Stage Position.vi"("Position"=w429, "error in"=w424, "VISA resource name in"=w425) -> ("error out"=w428:errorcluster)  [unwired: 2 out]
            n231 = local write "Stage Control Serial Error"(w428) -> ()
          }
          frame #2 {
            n232 = local write "Stage Moving"(FALSE ("Stage Moving")) -> ()
            n233 = case shown="True" "Cap 1 Flow ON" {
              frame False {
              }
              frame True {
                n234 = property on="Inject Pump 1" class="Bool (strict)"("Val(Sgnl)"=TRUE ("Value (Signaling)")) -> ()  [unwired: 2 in, 2 out]
              }
            }
            n235 = call <vilib>:"Beep.vi"() -> ()  [unwired: 3 in, 9 out]
          }
          frame #3 {
            n236 = property on="Sample Channel\nFlow" class="Bool (strict)"("Val(Sgnl)"=FALSE ("Value (Signaling)")) -> ()  [unwired: 2 in, 2 out]
            n237 = local read "Cap. 2 BD T1?\n(ADig T1, DNA T2)"() -> (w442:bool)
            n238 = case shown="True" w442 {
              tunnel: "Cap 1 T ON" -> [w444 w445]
              frame False {
                n239 = property on="Trap 1 (ON/OFF)" class="Bool (strict)"("Val(Sgnl)"=w444) -> ()  [unwired: 2 in, 2 out]
              }
              frame True {
                n240 = property on="Trap 2 (ON/OFF)" class="Bool (strict)"("Val(Sgnl)"=w445) -> ()  [unwired: 2 in, 2 out]
              }
            }
            n241 = property on="Got DNA bead" class="Bool"("Key Focus"=TRUE) -> ()  [unwired: 2 in, 2 out]
          }
        }
      }
      event "Move Cap. 2 (ADig Top)": Value Change {
        n242 = event-data() -> ()  [unwired: 1 in, 5 out]
        n243 = local write "Move Cap. 2 (ADig Top)"(FALSE ("Move Cap. 2 (ADig Left)")) -> ()
        n244 = flat-sequence {
          tunnel: w449 -> [w452]
          tunnel: w450 -> [w453]
          tunnel: [w453] -> w447
          tunnel: [w452] -> w446
          tunnel: w447 -> [w456]
          tunnel: w446 -> [w455]
          frame #0 {
            n245 = property on="Sample Channel\nFlow" class="Bool (strict)"("Val(Sgnl)"="Cap 2 Samp Flow ON") -> ()  [unwired: 2 in, 2 out]
          }
          frame #1 {
            w454 = FALSE ("Value (Signaling)")
            n246 = local read "Saved Stage Positions"() -> (w466:dbl[][])
            n247 = local write "Stage Moving"(TRUE ("Stage Moving")) -> ()
            n248 = Array Subset(array=w466, index (row)=1 ("index"), length (row)=1 ("length"), index (col)=1 ("index"), length (col)=3 ("length")) -> (w463:dbl[][])
            n249 = Reshape Array(w463, 3 ("dimension size")) -> (w461:dbl[])
            n250 = property on="Trap 1 (ON/OFF)" class="Bool (strict)"("Val(Sgnl)"=w454) -> ()  [unwired: 2 in, 2 out]
            n251 = property on="Trap 1 (ON/OFF)" class="Bool (strict)"("Val(Sgnl)"=w454) -> ()  [unwired: 2 in, 2 out]
            n252 = Array To Cluster(array=w461) -> (cluster=w460:cluster{"[0]":dbl, "[1]":dbl, "[2]":dbl})
            n253 = call "Set Stage Position.vi"("Position"=w460, "error in"=w455, "VISA resource name in"=w456) -> ("error out"=w459:errorcluster)  [unwired: 2 out]
            n254 = local write "Stage Control Serial Error"(w459) -> ()
          }
          frame #2 {
            n255 = local write "Stage Moving"(FALSE ("Stage Moving")) -> ()
            n256 = call <vilib>:"Beep.vi"() -> ()  [unwired: 3 in, 9 out]
            n257 = case shown="True" "Cap 2 Flow ON" {
              frame False {
              }
              frame True {
                n258 = property on="Inject Pump 3" class="Bool (strict)"("Val(Sgnl)"=TRUE ("Value (Signaling)")) -> ()  [unwired: 2 in, 2 out]
              }
            }
          }
          frame #3 {
            n259 = property on="Sample Channel\nFlow" class="Bool (strict)"("Val(Sgnl)"=FALSE ("Value (Signaling)")) -> ()  [unwired: 2 in, 2 out]
            n260 = case shown="False" "Cap. 2 BD T1?\n(ADig T1, DNA T2)" {
              tunnel: "Cap 2 T ON" -> [w475 w476]
              frame False {
                n261 = property on="Trap 2 (ON/OFF)" class="Bool (strict)"("Val(Sgnl)"=w475) -> ()  [unwired: 2 in, 2 out]
              }
              frame True {
                n262 = property on="Trap 1 (ON/OFF)" class="Bool (strict)"("Val(Sgnl)"=w476) -> ()  [unwired: 2 in, 2 out]
              }
            }
            n263 = property on="Got ADig bead" class="Bool"("Key Focus"=TRUE) -> ()  [unwired: 2 in, 2 out]
          }
        }
      }
      event "Initialize Blue Laser": Value Change {
        n264 = event-data() -> ()  [unwired: 1 in, 5 out]
        n265 = flat-sequence {
          tunnel: w477 -> [w496]
          frame #0 {
            n266 = Concatenate Strings("slmp ", "Blue Laser\nModulation\nPower (mW)") -> (w495:string)
            n267 = call "serial write macro.vi"("String"=w495, "Delay (ms)"="Delay (ms)", "VISA resource name"=w496) -> ("read buffer"=w484:string, "error out"=w485:errorcluster, "VISA resource name out"=w492:refnum<visa-resource-name>)
            n268 = local write "read blue buffer"(w484) -> ()
            n269 = local write "Blue Error Out"(w485) -> ()
            n270 = call "serial write macro.vi"("String"="sdmes 1", "Delay (ms)"="Delay (ms)", "VISA resource name"=w492) -> ("read buffer"=w482:string, "error out"=w483:errorcluster, "VISA resource name out"=w490:refnum<visa-resource-name>)
            n271 = local write "Blue Error Out"(w483) -> ()
            n272 = local write "read blue buffer"(w482) -> ()
            n273 = call "serial write macro.vi"("String"="sames 1", "Delay (ms)"="Delay (ms)", "VISA resource name"=w490) -> ("read buffer"=w479:string, "error out"=w481:errorcluster, "VISA resource name out"=w487:refnum<visa-resource-name>)
            n274 = local write "read blue buffer"(w479) -> ()
            n275 = local write "Blue Error Out"(w481) -> ()
            n276 = call "serial write macro.vi"("String"="l1", "Delay (ms)"="Delay (ms)", "VISA resource name"=w487) -> ("read buffer"=w478:string, "error out"=w480:errorcluster)  [unwired: 1 out]
            n277 = local write "read blue buffer"(w478) -> ()
            n278 = local write "Blue Error Out"(w480) -> ()
          }
          frame #1 {
            n279 = local write "Initialize Blue Laser"(FALSE ("Initialize")) -> ()
          }
        }
      }
      event "Blue Laser Modluation Mode": Value Change {
        # "Changes the type of modulation for the blue laser"
        n280 = event-data() -> ()  [unwired: 1 in, 5 out]
        n281 = case shown="\"Constant Power\"" "Blue Laser Modluation Mode" {
          tunnel: ["sdmes 1" w514 "sdmes 1" "sdmes 0"] -> w499
          tunnel: ["sames 1" "cp" "sames 0" "sames 1"] -> w498
          frame "Digital + Analog", Default {
          }
          frame "Constant Power" {
            n282 = local read "Blue Laser\nModulation\nPower (mW)"() -> (w517:string)
            n283 = Decimal String To Number(string=w517) -> (number=w513:i32)  [unwired: 2 in, 1 out]
            n284 = Divide(x=w513, y=1000) -> (x/y=w511:dbl)
            n285 = Number To Fractional String(number=w511) -> (F-format string=w512:string)  [unwired: 3 in]
            n286 = Concatenate Strings("p ", w512) -> (w514:string)
          }
          frame "Digital Only" {
          }
          frame "Analog Only" {
          }
        }
        n287 = local read "Delay (ms)"() -> (w508:i32)
        n288 = call "serial write macro.vi"("String"=w499, "Delay (ms)"=w508, "VISA resource name"=w505) -> ("read buffer"=w506:string, "error out"=w507:errorcluster, "VISA resource name out"=w500:refnum<visa-resource-name>)
        n289 = local write "read blue buffer"(w506) -> ()
        n290 = local write "Blue Error Out"(w507) -> ()
        n291 = local read "Delay (ms)"() -> (w503:i32)
        n292 = call "serial write macro.vi"("String"=w498, "Delay (ms)"=w503, "VISA resource name"=w500) -> ("read buffer"=w501:string, "error out"=w502:errorcluster)  [unwired: 1 out]
        n293 = local write "Blue Error Out"(w502) -> ()
        n294 = local write "read blue buffer"(w501) -> ()
      }
      event "Move in a Circle": Value Change {
        n295 = event-data() -> ()  [unwired: 1 in, 5 out]
        n296 = disable-structure shown="Disabled" {
          frame Disabled {
            # "converting distance (d) to angle (a)\na=arcsin(d/2r)"
            # "radius"
            # "radius"
            # "T1 Y"
            # "T1 X"
            n297 = local read "BD 1 Frequency 1 (MHz)"() -> (w532:dbl)
            n298 = local read "BD 2 Frequency 1 (MHz)"() -> (w531:dbl)
            n299 = Subtract(x=w531, y="Center Y Frequency (MHz)") -> (x-y=w533:dbl)
            n300 = node-c288() -> (w536:T23)  [unwired: 4 in]
            n301 = Absolute Value(x=w533) -> (abs(x)=w527:dbl)
            n302 = Multiply(x=w527, y=2) -> (x*y=w526:dbl)
            n303 = Divide(x="2D Motion Trap Separation (MHz)", y=w526) -> (x/y=w524:dbl)
            n304 = Inverse Sine(1:w524) -> (0:w528:dbl)
            n305 = Multiply(x=w528, y=2) -> (x*y=w523:dbl)
            n306 = timed-loop {
              tunnel: w527 -> [w542]
              timing: w536 -> [_]
              timing-out: [_] -> w535
              tunnel: w532 -> [_]
              tunnel: w531 -> [_]
              tunnel: w523 -> [w540]
              i -> [w556]
              stop <- "Stop Moving" stop-if-true
              # "r"
              # "r"
              # "r"
              # "r"
              # "\"omega*t\""
              # "Trap 2"
              # "Trap separation (radians)"
              # "Trap 1"
              # "Offset (starts\n at bottom of\n the circle)"
              # "\"t\""
              # "\"omega\""
              n307 = node-c288() -> (w558:i64)  [unwired: 1 in]
              n308 = Divide(x=w558, y=1000) -> (x/y=w557:dbl)
              n309 = Multiply(x=w557, y=w556) -> (x*y=w554:dbl)
              n310 = Multiply(x="2D Motion Frequency (Hz)", y=6.283185307179586) -> (x*y=w555:dbl)
              n311 = Multiply(x=w555, y=w554) -> (x*y=w538:dbl)
              n312 = Subtract(x=1.5707963267948966, y=w540) -> (x-y=w539:dbl)
              n313 = Subtract(x=w538, y=w539) -> (x-y=w547:dbl)
              n314 = Subtract(x=w538, y=1.5707963267948966) -> (x-y=w552:dbl)
              n315 = Cosine(x=w547) -> (cos(x)=w546:dbl)
              n316 = Sine(x=w547) -> (sin(x)=w545:dbl)
              n317 = Cosine(x=w552) -> (cos(x)=w551:dbl)
              n318 = Sine(x=w552) -> (sin(x)=w550:dbl)
              n319 = Multiply(x=w546, y=w542) -> (x*y=w544:dbl)
              n320 = Multiply(x=w545, y=w542) -> (x*y=w543:dbl)
              n321 = Multiply(x=w551, y=w542) -> (x*y=w549:dbl)
              n322 = Multiply(x=w550, y=w542) -> (x*y=w548:dbl)
              n323 = local write "BD 1 Frequency 1 (MHz)"(w549) -> ()
              n324 = local write "BD 2 Frequency 1 (MHz)"(w548) -> ()
              n325 = local write "BD 1 Frequency 2 (MHz)"(w544) -> ()
              n326 = local write "BD 2 Frequency 2 (MHz)"(w543) -> ()
              n327 = node-c288() -> ()  [unwired: 1 in, 1 out]
            }
            n328 = node-c288(w535) -> ()  [unwired: 1 out]
          }
          frame Enabled {
          }
        }
      }
      event "Blue Laser\nModulation\nPower (mW)": Value Change {
        n329 = event-data() -> ()  [unwired: 1 in, 5 out]
        n330 = local read "Blue Laser\nModulation\nPower (mW)"() -> (w568:string)
        n331 = local read "Blue Laser Modluation Mode"() -> (w569:string)
        n332 = case shown="\"Constant Power\"" w569 {
          tunnel: w568 -> [w575 w582]
          tunnel: [w574 w581] -> w567
          frame "Constant Power" {
            # "Different command to change constant power instead of modulation power"
            n333 = Decimal String To Number(string=w575) -> (offset past number=w580:i32)  [unwired: 2 in, 1 out]
            n334 = Divide(x=w580, y=1000) -> (x/y=w578:dbl)
            n335 = Number To Fractional String(number=w578) -> (F-format string=w576:string)  [unwired: 3 in]
            n336 = Concatenate Strings("p ", w576) -> (w574:string)
          }
          frame Default {
            n337 = Concatenate Strings("slmp ", w582) -> (w581:string)
          }
        }
        n338 = local read "Delay (ms)"() -> (w572:i32)
        n339 = call "serial write macro.vi"("String"=w567, "Delay (ms)"=w572, "VISA resource name"=w573) -> ("read buffer"=w571:string, "error out"=w570:errorcluster)  [unwired: 1 out]
        n340 = local write "Blue Error Out"(w570) -> ()
        n341 = local write "read blue buffer"(w571) -> ()
      }
      event "Send string\nto Blue Laser": Value Change {
        n342 = event-data() -> ()  [unwired: 1 in, 5 out]
        n343 = flat-sequence {
          tunnel: w584 -> [w589]
          frame #0 {
            n344 = local read "Delay (ms)"() -> (w586:i32)
            n345 = call "serial write macro.vi"("String"="command string", "Delay (ms)"=w586, "VISA resource name"=w589) -> ("read buffer"=w587:string, "error out"=→"Blue Error Out":errorcluster)  [unwired: 1 out]
            "read blue buffer" <- w587
            n346 = String Length(string=w587) -> (length=→"length":i32)
            "command string sent" <- "command string"
          }
          frame #1 {
            n347 = local write "Send string\nto Blue Laser"(FALSE ("Send string")) -> ()
          }
        }
      }
      event "Read Harvard": Value Change {
        n348 = event-data() -> ()  [unwired: 1 in, 5 out]
        n349 = Concatenate Strings("write buffer", "\r") -> (w596:string)
        n350 = VISA Write(VISA resource name=w594, write buffer=w596, error in (no error)=w593) -> (VISA resource name out=w605:refnum<visa-resource-name>, error out=w604:errorcluster)  [unwired: 1 out]
        n351 = stacked-sequence {
          tunnel: [w608] -> w603
          tunnel: w605 -> [w608]
          tunnel: w604 -> [w607]
          tunnel: [w607] -> w598
          frame #0 {
            n352 = Wait (ms)(milliseconds to wait=50) -> ()  [unwired: 1 out]
          }
        }
        n353 = property class="Instr"(reference=w603, error in=w598) -> (reference out=w602:refnum<visa-resource-name>, error out=w600:errorcluster, "Serial Settings:Number of Bytes at Serial Port"=w601:u32)
        "Serial Settings:Number of Bytes at Serial Port" <- w601
        n354 = VISA Read(VISA resource name=w602, byte count=w601, error in (no error)=w600) -> (read buffer=w599:string)  [unwired: 3 out]
        "read buffer" <- w599
        n355 = Fract/Exp String To Number(string=w599) -> ()  [unwired: 5 out]
      }
      event "+z", "-z": Value Change {
        n356 = event-data() -> ()  [unwired: 1 in, 5 out]
        n357 = flat-sequence {
          tunnel: w609 -> [w631]
          tunnel: w610 -> [w611]
          frame #0 {
            n358 = call "Read Stage Position.vi"("error in"=w631, "VISA resource name in"=w611) -> ("Current Position"=w616:cluster{dbl, dbl, dbl}, "error out"=w629:errorcluster, "VISA resource name out"=w630:refnum<visa-resource-name>)  [unwired: 1 out]
            n359 = local read "Saved Stage Positions"() -> (w640:dbl[][])
            n360 = Divide(x="z nudge increment (um)", y=1000.0) -> (x/y=w628:dbl)
            n361 = Boolean To (0,1)(Boolean="+z") -> (0, 1=w620:i16)
            n362 = Boolean To (0,1)(Boolean="-z") -> (0, 1=w621:i16)
            n363 = Array Subset(array=w640, index (row)=1 ("index"), length (row)=1 ("length"), index (col)=1 ("index"), length (col)=3 ("length")) -> (w637:dbl[][])
            n364 = Multiply(x=w620, y=w628) -> (x*y=w624:dbl)
            n365 = Multiply(x=w621, y=w628) -> (x*y=w622:dbl)
            n366 = Unbundle(w616) -> (w614:dbl, w613:dbl, w617:dbl)
            n367 = Negate(x=w622) -> (-x=w623:dbl)
            n368 = Reshape Array(w637, 3 ("dimension size")) -> (w635:dbl[])
            n369 = Add(x=w624, y=w623) -> (x+y=w625:dbl)
            n370 = Array To Cluster(array=w635) -> ()  [unwired: 1 out]
            n371 = Add(x=w625, y=w617) -> (x+y=w615:dbl)
            n372 = Bundle(cluster=w616, w614, w613, w615) -> (w612:cluster{dbl, dbl, dbl})
            n373 = call "Set Stage Position.vi"("Position"=w612, "error in"=w629, "VISA resource name in"=w630) -> ("error out"=w634:errorcluster)  [unwired: 2 out]
            n374 = local write "Stage Moving"(TRUE ("Stage Moving")) -> ()
            n375 = local write "Stage Control Serial Error"(w634) -> ()
          }
          frame #1 {
            n376 = local write "Stage Moving"(FALSE ("Stage Moving")) -> ()
            n377 = call <vilib>:"Beep.vi"() -> ()  [unwired: 3 in, 9 out]
          }
        }
      }
      event "Cal/Data Acq. Spot": Value Change {
        n378 = event-data() -> ()  [unwired: 1 in, 5 out]
        n379 = flat-sequence {
          tunnel: w649 -> [w653]
          tunnel: w650 -> [w654]
          tunnel: [w654] -> w646
          tunnel: [w653] -> w645
          tunnel: w646 -> [w659]
          tunnel: w645 -> [w658]
          tunnel: ["Cal @ (MHz)"] -> w643
          tunnel: [w663] -> w647
          tunnel: w643 -> [w663]
          tunnel: w647 -> [w672]
          tunnel: ["W/ Offset 1"] -> w644
          tunnel: w647 -> [w693]
          tunnel: w644 -> [w691]
          frame #0 {
            n380 = property on="Sample Channel\nFlow" class="Bool (strict)"("Val(Sgnl)"="Daq spot flow on") -> ()  [unwired: 2 in, 2 out]
            n381 = Wait (ms)(milliseconds to wait=u32 250) -> ()  [unwired: 1 out]
          }
          frame #1 {
            n382 = local read "Saved Stage Positions"() -> (w656:dbl[][])
            n383 = property on="Trap Delta (MHz)" class="DigNum (strict)"("Val(Sgnl)"="Cal @ (MHz)") -> ()  [unwired: 2 in, 2 out]
            n384 = local write "Stage Moving"(TRUE ("Stage Moving")) -> ()
            n385 = call "move to saved stage position.vi"("error in"=w658, "Stage VISA resource name in"=w659, "Position"="Cal Stage Position", "Saved Stage Positions"=w656) -> ("error out"=w657:errorcluster)  [unwired: 1 out]
            n386 = local write "Stage Control Serial Error"(w657) -> ()
          }
          frame #2 {
            n387 = local write "Stage Moving"(FALSE ("Stage Moving")) -> ()
            n388 = property on="Sample Channel\nFlow" class="Bool (strict)"("Val(Sgnl)"="Flow ON during cal?") -> ()  [unwired: 2 in, 2 out]
            n389 = call <vilib>:"Beep.vi"() -> ()  [unwired: 3 in, 9 out]
          }
          frame #3 {
            n390 = Wait (ms)(milliseconds to wait=u32 1000) -> ()  [unwired: 1 out]
          }
          frame #4 {
            n391 = property on="Save Calibration" class="Bool (strict)"("Val(Sgnl)"=TRUE ("Value (Signaling)")) -> ()  [unwired: 2 in, 2 out]
          }
          frame #5 {
            n392 = Wait (ms)(milliseconds to wait=u32 2000) -> ()  [unwired: 1 out]
          }
          frame #6 {
            # "Check to see if \nsaving done"
            n393 = while {
              stop <- w668 stop-if-true
              n394 = local read "Saving..."() -> (w669:bool)
              n395 = Wait (ms)(milliseconds to wait=u32 100) -> ()  [unwired: 1 out]
              n396 = Not(x=w669) -> (.not. x?=w668:bool)
            }
          }
          frame #7 {
            n397 = case shown="True" "W/ Offset 1" {
              tunnel: w672 -> [_ w673]
              frame False {
              }
              frame True {
                n398 = stacked-sequence {
                  tunnel: w673 -> [_ _ _ _ _ _ _ w690]
                  frame #0 {
                    n399 = property on="Trap Delta (MHz)" class="DigNum (strict)"("Val(Sgnl)"="Offset 1 Start (MHz)") -> ()  [unwired: 2 in, 2 out]
                    n400 = Replace Array Subset(array=u32[] [0] ("Index Values"), new element="Offset 1 Set", index=0) -> (w674:u32[])